vi "Dresden R2R Sputter 03.02.2018 IY24.vi"() -> ()   [LabVIEW 2009] (continued)
                                n22591 = Wait Until Next ms Multiple(millisecond multiple=u32 200) -> ()  [unwired: 1 out]
                                n22592 = local write "Ch4_Tp_bv_do"(FALSE ("Ch1_Ch_cc_on_off_di")) -> ()
                                }
                                }
                                n22593 = local read "Semi"() -> (w21868:bool)
                                n22594 = Or(x=w21867, y=w21868) -> (x .or. y?=w21866:bool)
                                }
                                }
                                frame #1 {
                                }
                                }
                                }
                                frame #1 {
                                n22595 = local read "Semi"() -> (w21879:bool)
                                n22596 = case shown="False" w21879 {
                                frame #0 {
                                n22597 = Wait (ms)(milliseconds to wait=u32 1000) -> ()  [unwired: 1 out]
                                n22598 = local write "Ch4_Sd6"(TRUE ("Ch1_Sd5")) -> ()
                                }
                                frame #1 {
                                }
                                }
                                }
                                }
                                }
                                frame #1 {
                                }
                                }
                              }
                              frame #6 {
                                # "STOP MP"
                                n22599 = local read "Semi"() -> (w21882:bool)
                                n22600 = case shown="False" w21882 {
                                frame #0 {
                                n22601 = stacked-sequence {
                                frame #0 {
                                n22602 = local read "Semi"() -> (w21883:bool)
                                n22603 = case shown="False" w21883 {
                                frame #0 {
                                n22604 = while {
                                i -> [w21889]
                                stop <- w21884 stop-if-true
                                n22605 = Greater?(x=w21889, y=25) -> (0:w21888:bool)
                                n22606 = case shown="True" w21888 {
                                frame #0 {
                                }
                                frame #1 {
                                n22607 = local write "Error Message"("Shut Down Process  cancelled\nbecause  MP not closed.\nPlease check MP4  connections." ("Error Message")) -> ()
                                n22608 = local write "Semi"(TRUE ("Semi")) -> ()
                                }
                                }
                                n22609 = local read "Ch4_Mp_di"() -> (w21887:bool)
                                n22610 = case shown="True" w21887 {
                                tunnel: [TRUE FALSE] -> w21885
                                frame #0 {
                                }
                                frame #1 {
                                n22611 = Wait Until Next ms Multiple(millisecond multiple=u32 200) -> ()  [unwired: 1 out]
                                n22612 = local write "Ch4_Mp_do"(FALSE ("Ch1_Ch_cc_on_off_di")) -> ()
                                }
                                }
                                n22613 = local read "Semi"() -> (w21886:bool)
                                n22614 = Or(x=w21885, y=w21886) -> (x .or. y?=w21884:bool)
                                }
                                }
                                frame #1 {
                                }
                                }
                                }
                                frame #1 {
                                n22615 = local read "Semi"() -> (w21897:bool)
                                n22616 = case shown="False" w21897 {
                                frame #0 {
                                n22617 = local write "Ch4_Sd7"(TRUE ("Ch1_Sd6")) -> ()
                                n22618 = Wait (ms)(milliseconds to wait=u32 1000) -> ()  [unwired: 1 out]
                                }
                                frame #1 {
                                }
                                }
                                }
                                }
                                }
                                frame #1 {
                                }
                                }
                              }
                              frame #7 {
                                # "PL-VBV OPEN  & CHECK"
                                n22619 = local read "Semi"() -> (w21900:bool)
                                n22620 = case shown="False" w21900 {
                                frame #0 {
                                n22621 = stacked-sequence {
                                frame #0 {
                                n22622 = local read "Semi"() -> (w21901:bool)
                                n22623 = case shown="False" w21901 {
                                frame #0 {
                                n22624 = local write "Ch4_Pl_atm_do"(FALSE ("Ch1_Pl_atm_do")) -> ()
                                n22625 = Wait Until Next ms Multiple(millisecond multiple=u32 2000) -> ()  [unwired: 1 out]
                                }
                                frame #1 {
                                }
                                }
                                }
                                frame #1 {
                                n22626 = local read "Semi"() -> (w21904:bool)
                                n22627 = case shown="False" w21904 {
                                frame #0 {
                                n22628 = while {
                                i -> [w21910]
                                stop <- w21906 stop-if-true
                                n22629 = Greater?(x=w21910, y=50) -> (0:w21909:bool)
                                n22630 = case shown="True" w21909 {
                                frame #0 {
                                }
                                frame #1 {
                                n22631 = local write "Error Message"("Shut Down Process  cancelled\nbecause  PL-VBV not opened.\nPlease check  PL-VBV4 connections." ("Error Message")) -> ()
                                n22632 = local write "Semi"(TRUE ("Semi")) -> ()
                                }
                                }
                                n22633 = local read "Ch4_Pl_atm_di"() -> (w21905:bool)
                                n22634 = case shown="False" w21905 {
                                tunnel: [w21912 TRUE] -> w21907
                                frame #0 {
                                n22635 = local read "Ch4_Pl_vbv_di"() -> (w21913:bool)
                                n22636 = case shown="False" w21913 {
                                tunnel: [FALSE TRUE] -> w21912
                                frame #0 {
                                n22637 = Wait Until Next ms Multiple(millisecond multiple=u32 500) -> ()  [unwired: 1 out]
                                n22638 = local write "Ch4_Pl_vbv_do"(TRUE ("Ch1_Ch_cc_on_off_di")) -> ()
                                }
                                frame #1 {
                                }
                                }
                                }
                                frame #1 {
                                n22639 = Wait Until Next ms Multiple(millisecond multiple=u32 500) -> ()  [unwired: 1 out]
                                }
                                }
                                n22640 = local read "Semi"() -> (w21908:bool)
                                n22641 = Or(x=w21907, y=w21908) -> (x .or. y?=w21906:bool)
                                }
                                }
                                frame #1 {
                                }
                                }
                                }
                                frame #2 {
                                n22642 = local read "Semi"() -> (w21922:bool)
                                n22643 = case shown="False" w21922 {
                                frame #0 {
                                n22644 = local write "Ch4_Sd8"(FALSE ("Ch1_Sd8")) -> ()
                                n22645 = Wait (ms)(milliseconds to wait=u32 1000) -> ()  [unwired: 1 out]
                                }
                                frame #1 {
                                }
                                }
                                }
                                }
                                }
                                frame #1 {
                                }
                                }
                              }
                              frame #8 {
                                # "PL-VBV CLOSE  & CHECK"
                                n22646 = local read "Semi"() -> (w21925:bool)
                                n22647 = case shown="False" w21925 {
                                frame #0 {
                                n22648 = stacked-sequence {
                                frame #0 {
                                n22649 = local read "Semi"() -> (w21926:bool)
                                n22650 = case shown="False" w21926 {
                                frame #0 {
                                n22651 = while {
                                i -> [w21932]
                                stop <- w21928 stop-if-true
                                n22652 = Greater?(x=w21932, y=50) -> (0:w21931:bool)
                                n22653 = case shown="True" w21931 {
                                frame #0 {
                                }
                                frame #1 {
                                n22654 = local write "Error Message"("Shut Down Process  cancelled\nbecause  PL-VBV not closed.\nPlease check PL-VBV4  connections." ("Error Message")) -> ()
                                n22655 = local write "Semi"(TRUE ("Semi")) -> ()
                                }
                                }
                                n22656 = local read "Ch4_Pl_atm_di"() -> (w21927:bool)
                                n22657 = case shown="True" w21927 {
                                tunnel: [FALSE w21936] -> w21929
                                frame #0 {
                                n22658 = Wait Until Next ms Multiple(millisecond multiple=u32 500) -> ()  [unwired: 1 out]
                                }
                                frame #1 {
                                n22659 = local read "Ch4_Pl_vbv_di"() -> (w21937:bool)
                                n22660 = case shown="True" w21937 {
                                tunnel: [TRUE FALSE] -> w21936
                                frame #0 {
                                }
                                frame #1 {
                                n22661 = Wait Until Next ms Multiple(millisecond multiple=u32 500) -> ()  [unwired: 1 out]
                                n22662 = local write "Ch4_Pl_vbv_do"(FALSE ("Ch1_Ch_cc_on_off_di")) -> ()
                                }
                                }
                                }
                                }
                                n22663 = local read "Semi"() -> (w21930:bool)
                                n22664 = Or(x=w21929, y=w21930) -> (x .or. y?=w21928:bool)
                                }
                                }
                                frame #1 {
                                }
                                }
                                }
                                frame #1 {
                                n22665 = local read "Semi"() -> (w21944:bool)
                                n22666 = case shown="False" w21944 {
                                frame #0 {
                                n22667 = local write "Ch4_Sd 9"(TRUE ("Ch1_Sd11")) -> ()
                                n22668 = Wait (ms)(milliseconds to wait=u32 1000) -> ()  [unwired: 1 out]
                                }
                                frame #1 {
                                }
                                }
                                }
                                }
                                }
                                frame #1 {
                                }
                                }
                              }
                              frame #9 {
                                # "WAIT DECELARATING TP"
                                n22669 = local read "Semi"() -> (w21947:bool)
                                n22670 = case shown="False" w21947 {
                                frame #0 {
                                n22671 = stacked-sequence {
                                frame #0 {
                                n22672 = local read "Semi"() -> (w21948:bool)
                                n22673 = case shown="False" w21948 {
                                frame #0 {
                                n22674 = while {
                                i -> [w21954]
                                stop <- w21950 stop-if-true
                                n22675 = Greater?(x=w21954, y=1500) -> (0:w21953:bool)
                                n22676 = case shown="True" w21953 {
                                frame #0 {
                                }
                                frame #1 {
                                n22677 = local write "Error Message"("Shut Down Process  cancelled\nbecause TP not decelarating.\nPlease check TP4  connections." ("Error Message")) -> ()
                                n22678 = local write "Semi"(TRUE ("Semi")) -> ()
                                }
                                }
                                n22679 = local read "Yes 4"() -> (w21949:bool)
                                n22680 = case shown="True" w21949 {
                                tunnel: [TRUE w21960] -> w21951
                                frame #0 {
                                }
                                frame #1 {
                                n22681 = local read "Tp4_speed_gui"() -> (w21958:i32)
                                n22682 = Less?(x=w21958, y="Tp4_safety_speed") -> (x < y?=w21957:bool)
                                n22683 = case shown="False" w21957 {
                                tunnel: [FALSE TRUE] -> w21960
                                frame #0 {
                                n22684 = Wait Until Next ms Multiple(millisecond multiple=u32 500) -> ()  [unwired: 1 out]
                                }
                                frame #1 {
                                }
                                }
                                }
                                }
                                n22685 = local read "Semi"() -> (w21952:bool)
                                n22686 = Or(x=w21951, y=w21952) -> (x .or. y?=w21950:bool)
                                }
                                }
                                frame #1 {
                                }
                                }
                                }
                                frame #1 {
                                n22687 = local read "Semi"() -> (w21966:bool)
                                n22688 = case shown="False" w21966 {
                                frame #0 {
                                n22689 = Wait (ms)(milliseconds to wait=u32 1000) -> ()  [unwired: 1 out]
                                n22690 = local write "Ch4_Sd10"(TRUE ("Ch1_Sd3")) -> ()
                                }
                                frame #1 {
                                }
                                }
                                }
                                }
                                }
                                frame #1 {
                                }
                                }
                              }
                              frame #10 {
                                # "CH-VBV OPEN  & CHECK"
                                n22691 = local read "Yes 4"() -> (w21969:bool)
                                n22692 = case shown="True" w21969 {
                                frame #0 {
                                }
                                frame #1 {
                                n22693 = local read "Semi"() -> (w21970:bool)
                                n22694 = case shown="False" w21970 {
                                frame #0 {
                                n22695 = stacked-sequence {
                                frame #0 {
                                n22696 = local read "Semi"() -> (w21971:bool)
                                n22697 = case shown="False" w21971 {
                                frame #0 {
                                n22698 = local write "Ch4_Ch_atm_do"(FALSE ("Ch1_Pl_atm_do")) -> ()
                                n22699 = Wait Until Next ms Multiple(millisecond multiple=u32 2000) -> ()  [unwired: 1 out]
                                }
                                frame #1 {
                                }
                                }
                                }
                                frame #1 {
                                n22700 = local read "Semi"() -> (w21974:bool)
                                n22701 = case shown="False" w21974 {
                                frame #0 {
                                n22702 = while {
                                i -> [w21980]
                                stop <- w21976 stop-if-true
                                n22703 = Greater?(x=w21980, y=50) -> (0:w21979:bool)
                                n22704 = case shown="True" w21979 {
                                frame #0 {
                                }
                                frame #1 {
                                n22705 = local write "Error Message"("Shut Down Process  cancelled\nbecause  CH-VBV not opened.\nPlease check  CH-VBV4  connections." ("Error Message")) -> ()
                                n22706 = local write "Semi"(TRUE ("Semi")) -> ()
                                }
                                }
                                n22707 = local read "Ch4_Ch_atm_di"() -> (w21975:bool)
                                n22708 = case shown="False" w21975 {
                                tunnel: [w21982 TRUE] -> w21977
                                frame #0 {
                                n22709 = local read "Ch4_Ch_vbv_di"() -> (w21983:bool)
                                n22710 = case shown="False" w21983 {
                                tunnel: [FALSE TRUE] -> w21982
                                frame #0 {
                                n22711 = Wait Until Next ms Multiple(millisecond multiple=u32 200) -> ()  [unwired: 1 out]
                                n22712 = local write "Ch4_Ch_vbv_do"(TRUE ("Ch1_Ch_cc_on_off_di")) -> ()
                                }
                                frame #1 {
                                }
                                }
                                }
                                frame #1 {
                                }
                                }
                                n22713 = local read "Semi"() -> (w21978:bool)
                                n22714 = Or(x=w21977, y=w21978) -> (x .or. y?=w21976:bool)
                                }
                                }
                                frame #1 {
                                }
                                }
                                }
                                frame #2 {
                                n22715 = local read "Semi"() -> (w21991:bool)
                                n22716 = case shown="False" w21991 {
                                frame #0 {
                                n22717 = local write "Ch4_Sd11"(TRUE ("Ch1_Sd9")) -> ()
                                n22718 = Wait (ms)(milliseconds to wait=u32 1000) -> ()  [unwired: 1 out]
                                }
                                frame #1 {
                                }
                                }
                                }
                                }
                                }
                                frame #1 {
                                }
                                }
                                }
                                }
                              }
                              frame #11 {
                                # "CH-VBV CLOSE &  CHECK"
                                n22719 = local read "Yes 4"() -> (w21994:bool)
                                n22720 = case shown="True" w21994 {
                                frame #0 {
                                }
                                frame #1 {
                                n22721 = local read "Semi"() -> (w21995:bool)
                                n22722 = case shown="False" w21995 {
                                frame #0 {
                                n22723 = stacked-sequence {
                                frame #0 {
                                n22724 = local read "Semi"() -> (w21996:bool)
                                n22725 = case shown="False" w21996 {
                                frame #0 {
                                n22726 = while {
                                i -> [w22004]
                                stop <- w22000 stop-if-true
                                n22727 = Greater?(x=w22004, y=50) -> (0:w22003:bool)
                                n22728 = case shown="True" w22003 {
                                frame #0 {
                                }
                                frame #1 {
                                n22729 = local write "Error Message"("Shut Down Process  cancelled\nbecause  CH-VBV  not closed.\nPlease check CH-VBV4  connections." ("Error Message")) -> ()
                                n22730 = local write "Semi"(TRUE ("Semi")) -> ()
                                }
                                }
                                n22731 = local read "Tp4_speed_gui"() -> (w21998:i32)
                                n22732 = Greater Or Equal?(x=w21998, y=u64 100) -> (x >= y?=w21997:bool)
                                n22733 = case shown="True" w21997 {
                                tunnel: [TRUE w22007] -> w22001
                                frame #0 {
                                }
                                frame #1 {
                                n22734 = local read "Ch4_Ch_vbv_di"() -> (w22008:bool)
                                n22735 = case shown="True" w22008 {
                                tunnel: [TRUE FALSE] -> w22007
                                frame #0 {
                                }
                                frame #1 {
                                n22736 = Wait Until Next ms Multiple(millisecond multiple=u32 500) -> ()  [unwired: 1 out]
                                n22737 = local write "Ch4_Ch_vbv_do"(FALSE ("Ch1_Ch_cc_on_off_di")) -> ()
                                }
                                }
                                }
                                }
                                n22738 = local read "Semi"() -> (w22002:bool)
                                n22739 = Or(x=w22001, y=w22002) -> (x .or. y?=w22000:bool)
                                }
                                }
                                frame #1 {
                                }
                                }
                                }
                                frame #1 {
                                n22740 = local read "Semi"() -> (w22015:bool)
                                n22741 = case shown="False" w22015 {
                                frame #0 {
                                n22742 = local write "Ch4_Sd12"(TRUE ("Ch1_Sd13")) -> ()
                                n22743 = Wait (ms)(milliseconds to wait=u32 1000) -> ()  [unwired: 1 out]
                                }
                                frame #1 {
                                }
                                }
                                }
                                frame #2 {
                                n22744 = local read "Semi"() -> (w22018:bool)
                                n22745 = case shown="False" w22018 {
                                frame #0 {
                                n22746 = Wait (ms)(milliseconds to wait=u32 3000) -> ()  [unwired: 1 out]
                                }
                                frame #1 {
                                }
                                }
                                }
                                }
                                }
                                frame #1 {
                                }
                                }
                                }
                                }
                              }
                              frame #12 {
                                # "CH-VBV OPEN &  CHECK"
                                n22747 = local read "Yes 4"() -> (w22020:bool)
                                n22748 = case shown="True" w22020 {
                                frame #0 {
                                }
                                frame #1 {
                                n22749 = local read "Semi"() -> (w22021:bool)
                                n22750 = case shown="False" w22021 {
                                frame #0 {
                                n22751 = stacked-sequence {
                                frame #0 {
                                n22752 = local read "Semi"() -> (w22022:bool)
                                n22753 = case shown="False" w22022 {
                                frame #0 {
                                n22754 = while {
                                i -> [w22028]
                                stop <- w22024 stop-if-true
                                n22755 = Greater?(x=w22028, y=200) -> (0:w22027:bool)
                                n22756 = case shown="True" w22027 {
                                frame #0 {
                                }
                                frame #1 {
                                n22757 = local write "Error Message"("Shut Down Process  cancelled\nbecause  CH-VBV  not opened.\nPlease check CH-VBV4  connections." ("Error Message")) -> ()
                                n22758 = local write "Semi"(TRUE ("Semi")) -> ()
                                }
                                }
                                n22759 = local read "Ch4_Ch_vbv_di"() -> (w22023:bool)
                                n22760 = case shown="False" w22023 {
                                tunnel: [FALSE TRUE] -> w22025
                                frame #0 {
                                n22761 = local write "Ch4_Ch_vbv_do"(TRUE ("Ch1_Ch_cc_on_off_di")) -> ()
                                n22762 = Wait Until Next ms Multiple(millisecond multiple=u32 500) -> ()  [unwired: 1 out]
                                }
                                frame #1 {
                                }
                                }
                                n22763 = local read "Semi"() -> (w22026:bool)
                                n22764 = Or(x=w22025, y=w22026) -> (x .or. y?=w22024:bool)
                                }
                                }
                                frame #1 {
                                }
                                }
                                }
                                frame #1 {
                                n22765 = local read "Semi"() -> (w22036:bool)
                                n22766 = case shown="False" w22036 {
                                frame #0 {
                                n22767 = Wait (ms)(milliseconds to wait=u32 1000) -> ()  [unwired: 1 out]
                                n22768 = local write "Ch4_Sd13"(TRUE ("Ch1_Sd12")) -> ()
                                }
                                frame #1 {
                                }
                                }
                                }
                                }
                                }
                                frame #1 {
                                }
                                }
                                }
                                }
                              }
                              frame #13 {
                                # "TRNS GV-BP OPEN"
                                n22769 = local read "Yes 4"() -> (w22039:bool)
                                n22770 = case shown="True" w22039 {
                                frame #0 {
                                }
                                frame #1 {
                                n22771 = local read "Semi"() -> (w22040:bool)
                                n22772 = case shown="False" w22040 {
                                frame #0 {
                                n22773 = stacked-sequence {
                                frame #0 {
                                n22774 = local read "Semi"() -> (w22041:bool)
                                n22775 = case shown="False" w22041 {
                                frame #0 {
                                n22776 = while {
                                i -> [w22049]
                                stop <- w22046 stop-if-true
                                n22777 = Greater?(x=w22049, y=800) -> (0:w22048:bool)
                                n22778 = case shown="True" w22048 {
                                frame #0 {
                                }
                                frame #1 {
                                n22779 = local write "Error Message"("Shut Down process was cancelled.\nPlease check Trns GV-BP\n connections." ("Error Message")) -> ()
                                n22780 = local write "Semi"(TRUE ("Semi")) -> ()
                                }
                                }
                                n22781 = local read "Ch4pressure"() -> (w22044:dbl)
                                n22782 = Greater Or Equal?(x=w22044, y=700.0) -> (x >= y?=w22042:bool)
                                n22783 = case shown="True" w22042 {
                                tunnel: [FALSE w22053] -> w22045
                                frame #0 {
                                n22784 = Wait Until Next ms Multiple(millisecond multiple=u32 500) -> ()  [unwired: 1 out]
                                }
                                frame #1 {
                                n22785 = local read "Ch4_Trns_gv_bp_di"() -> (w22054:bool)
                                n22786 = case shown="False" w22054 {
                                tunnel: [FALSE TRUE] -> w22053
                                frame #0 {
                                n22787 = local write "Ch4_Trns_gv_bp_do"(TRUE ("Ch1_Trns_gv_bp2_do")) -> ()
                                n22788 = Wait Until Next ms Multiple(millisecond multiple=u32 500) -> ()  [unwired: 1 out]
                                }
                                frame #1 {
                                }
                                }
                                }
                                }
                                n22789 = local read "Semi"() -> (w22047:bool)
                                n22790 = Or(x=w22045, y=w22047) -> (x .or. y?=w22046:bool)
                                }
                                }
                                frame #1 {
                                }
                                }
                                }
                                frame #1 {
                                n22791 = local read "Semi"() -> (w22061:bool)
                                n22792 = case shown="False" w22061 {
                                frame #0 {
                                n22793 = local write "Ch4_Sd14"(TRUE ("Ch4_Sd0 14")) -> ()
                                n22794 = Wait (ms)(milliseconds to wait=u32 1000) -> ()  [unwired: 1 out]
                                }
                                frame #1 {
                                }
                                }
                                }
                                frame #2 {
                                n22795 = local read "Semi"() -> (w22064:bool)
                                n22796 = case shown="False" w22064 {
                                frame #0 {
                                n22797 = Wait (ms)(milliseconds to wait=u32 2000) -> ()  [unwired: 1 out]
                                }
                                frame #1 {
                                }
                                }
                                }
                                }
                                }
                                frame #1 {
                                }
                                }
                                }
                                }
                              }
                              frame #14 {
                                # "CH-ATM OPEN &  CHECK"
                                n22798 = local read "Yes 4"() -> (w22066:bool)
                                n22799 = case shown="True" w22066 {
                                frame #0 {
                                }
                                frame #1 {
                                n22800 = local read "Semi"() -> (w22067:bool)
                                n22801 = case shown="False" w22067 {
                                frame #0 {
                                n22802 = stacked-sequence {
                                frame #0 {
                                n22803 = local read "Semi"() -> (w22068:bool)
                                n22804 = case shown="False" w22068 {
                                frame #0 {
                                n22805 = while {
                                i -> [w22074]
                                stop <- w22071 stop-if-true
                                n22806 = Greater?(x=w22074, y=1700) -> (0:w22073:bool)
                                n22807 = case shown="True" w22073 {
                                frame #0 {
                                }
                                frame #1 {
                                n22808 = local write "Error Message"("Shut Down process was cancelled.\nPlease check Chamber \nvacuum connections." ("Error Message")) -> ()
                                n22809 = local write "Semi"(TRUE ("Semi")) -> ()
                                }
                                }
                                n22810 = local read "Ch4_Ch_atm_di"() -> (w22070:bool)
                                n22811 = case shown="False" w22070 {
                                tunnel: [FALSE TRUE] -> w22069
                                frame #0 {
                                n22812 = Wait Until Next ms Multiple(millisecond multiple=u32 500) -> ()  [unwired: 1 out]
                                }
                                frame #1 {
                                }
                                }
                                n22813 = local read "Semi"() -> (w22072:bool)
                                n22814 = Or(x=w22069, y=w22072) -> (x .or. y?=w22071:bool)
                                }
                                }
                                frame #1 {
                                }
                                }
                                }
                                frame #1 {
                                n22815 = local read "Semi"() -> (w22081:bool)
                                n22816 = case shown="False" w22081 {
                                frame #0 {
                                n22817 = Wait (ms)(milliseconds to wait=u32 1000) -> ()  [unwired: 1 out]
                                n22818 = local write "Ch4_Sd15"(TRUE ("Ch1_Sd10")) -> ()
                                }
                                frame #1 {
                                }
                                }
                                }
                                frame #2 {
                                n22819 = local read "Semi"() -> (w22084:bool)
                                n22820 = case shown="False" w22084 {
                                frame #0 {
                                n22821 = Wait (ms)(milliseconds to wait=u32 2000) -> ()  [unwired: 1 out]
                                }
                                frame #1 {
                                }
                                }
                                }
                                }
                                }
                                frame #1 {
                                }
                                }
                                }
                                }
                              }
                              frame #15 {
                                # "TRNS GV-BP close"
                                n22822 = local read "Semi"() -> (w22086:bool)
                                n22823 = case shown="False" w22086 {
                                frame #0 {
                                n22824 = stacked-sequence {
                                frame #0 {
                                n22825 = local read "Semi"() -> (w22087:bool)
                                n22826 = case shown="False" w22087 {
                                frame #0 {
                                n22827 = while {
                                i -> [w22093]
                                stop <- w22089 stop-if-true
                                n22828 = Greater?(x=w22093, y=50) -> (0:w22092:bool)
                                n22829 = case shown="True" w22092 {
                                frame #0 {
                                }
                                frame #1 {
                                n22830 = local write "Error Message"("Shut Down Process  cancelled\nbecause  Trns-GV-BP  not closed.\nPlease check Trns-GV-BP connections." ("Error Message")) -> ()
                                n22831 = local write "Semi"(TRUE ("Semi")) -> ()
                                }
                                }
                                n22832 = local read "Ch4_Trns_gv_bp_di"() -> (w22088:bool)
                                n22833 = case shown="True" w22088 {
                                tunnel: [TRUE FALSE] -> w22090
                                frame #0 {
                                }
                                frame #1 {
                                n22834 = Wait Until Next ms Multiple(millisecond multiple=u32 500) -> ()  [unwired: 1 out]
                                n22835 = local write "Ch4_Trns_gv_bp_do"(FALSE ("Ch1_Ch_cc_on_off_di")) -> ()
                                }
                                }
                                n22836 = local read "Semi"() -> (w22091:bool)
                                n22837 = Or(x=w22090, y=w22091) -> (x .or. y?=w22089:bool)
                                }
                                }
                                frame #1 {
                                }
                                }
                                }
                                frame #1 {
                                n22838 = local read "Semi"() -> (w22101:bool)
                                n22839 = case shown="False" w22101 {
                                frame #0 {
                                n22840 = local write "Ch4_Sd16"(TRUE ("Ch1_Sd10 3")) -> ()
                                n22841 = Wait (ms)(milliseconds to wait=u32 1000) -> ()  [unwired: 1 out]
                                }
                                frame #1 {
                                }
                                }
                                }
                                }
                                }
                                frame #1 {
                                }
                                }
                              }
                              frame #16 {
                                # "CH-VBV CLOSE &  CHECK"
                                n22842 = local read "Yes 4"() -> (w22104:bool)
                                n22843 = case shown="True" w22104 {
                                frame #0 {
                                }
                                frame #1 {
                                n22844 = local read "Semi"() -> (w22105:bool)
                                n22845 = case shown="False" w22105 {
                                frame #0 {
                                n22846 = stacked-sequence {
                                frame #0 {
                                n22847 = local read "Semi"() -> (w22106:bool)
                                n22848 = case shown="False" w22106 {
                                frame #0 {
                                n22849 = while {
                                i -> [w22116]
                                stop <- w22112 stop-if-true
                                n22850 = Greater?(x=w22116, y=50) -> (0:w22115:bool)
                                n22851 = case shown="True" w22115 {
                                frame #0 {
                                }
                                frame #1 {
                                n22852 = local write "Error Message"("Shut Down Process  cancelled\nbecause  CH-VBV  not closed.\nPlease check CH-VBV4 connections." ("Error Message")) -> ()
                                n22853 = local write "Semi"(TRUE ("Semi")) -> ()
                                }
                                }
                                n22854 = local read "Tp4_speed_gui"() -> (w22110:i32)
                                n22855 = local read "Yes 4"() -> (w22109:bool)
                                n22856 = Greater Or Equal?(x=w22110, y=u64 100) -> (x >= y?=w22108:bool)
                                n22857 = And(x=w22109, y=w22108) -> (x .and. y?=w22107:bool)
                                n22858 = case shown="True" w22107 {
                                tunnel: [TRUE w22119] -> w22113
                                frame #0 {
                                }
                                frame #1 {
                                n22859 = local read "Ch4_Ch_vbv_di"() -> (w22120:bool)
                                n22860 = case shown="True" w22120 {
                                tunnel: [TRUE FALSE] -> w22119
                                frame #0 {
                                }
                                frame #1 {
                                n22861 = Wait Until Next ms Multiple(millisecond multiple=u32 500) -> ()  [unwired: 1 out]
                                n22862 = local write "Ch4_Ch_vbv_do"(FALSE ("Ch1_Ch_cc_on_off_di")) -> ()
                                }
                                }
                                }
                                }
                                n22863 = local read "Semi"() -> (w22114:bool)
                                n22864 = Or(x=w22113, y=w22114) -> (x .or. y?=w22112:bool)
                                }
                                }
                                frame #1 {
                                }
                                }
                                }
                                frame #1 {
                                n22865 = local read "Semi"() -> (w22127:bool)
                                n22866 = case shown="False" w22127 {
                                frame #0 {
                                n22867 = local write "Ch4_Sd17"(TRUE ("Ch1_Sd10 2")) -> ()
                                n22868 = Wait (ms)(milliseconds to wait=u32 1000) -> ()  [unwired: 1 out]
                                }
                                frame #1 {
                                }
                                }
                                }
                                frame #2 {
                                n22869 = local read "Semi"() -> (w22130:bool)
                                n22870 = case shown="False" w22130 {
                                frame #0 {
                                n22871 = Wait (ms)(milliseconds to wait=u32 3000) -> ()  [unwired: 1 out]
                                }
                                frame #1 {
                                }